vi "IR Opo Main.vi"() -> ()   [LabVIEW 2016] (continued)
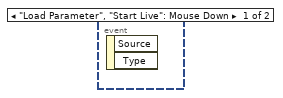
[diagram p2: hidden frame]
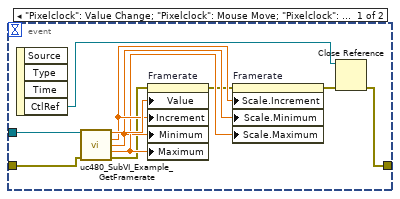
[diagram p3: hidden frame]
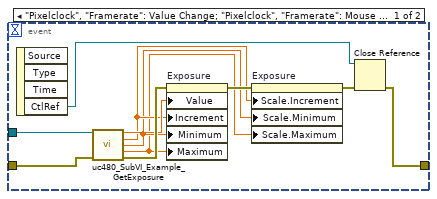
[diagram p4: hidden frame]
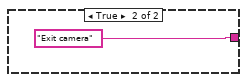
[diagram p5: hidden frame]
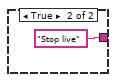
[diagram p6: hidden frame]
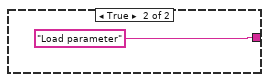
[diagram p7: hidden frame]
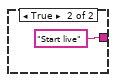
[diagram p8: hidden frame]
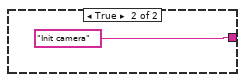
[diagram p9: hidden frame]
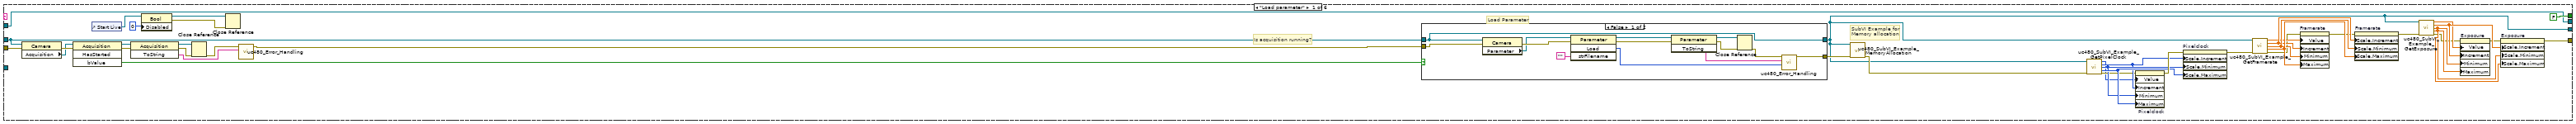
[diagram p10: hidden frame]
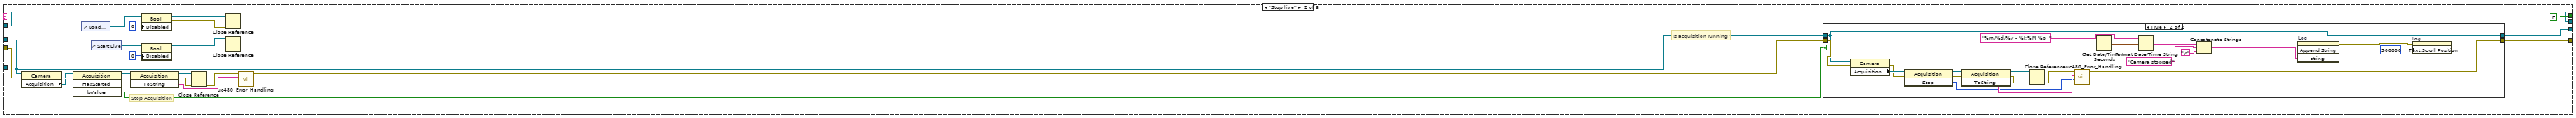
[diagram p12: hidden frame]
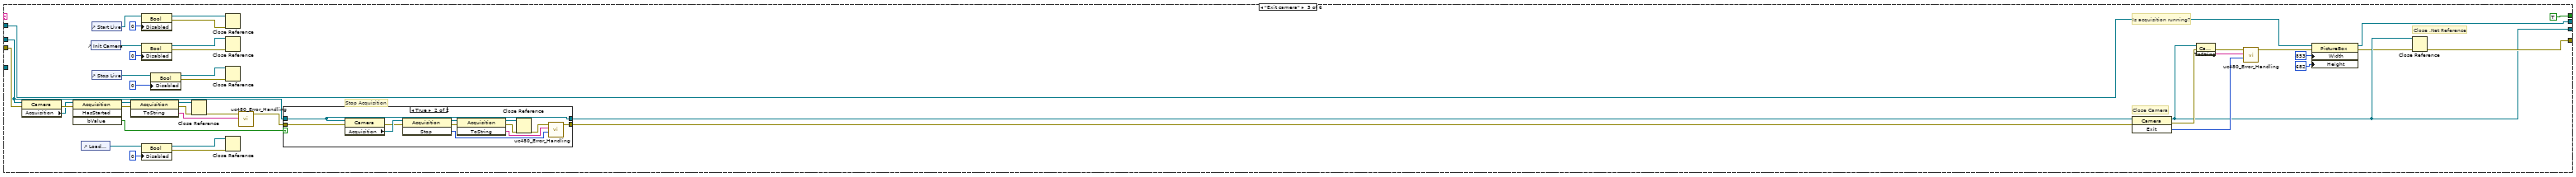
[diagram p14: hidden frame]
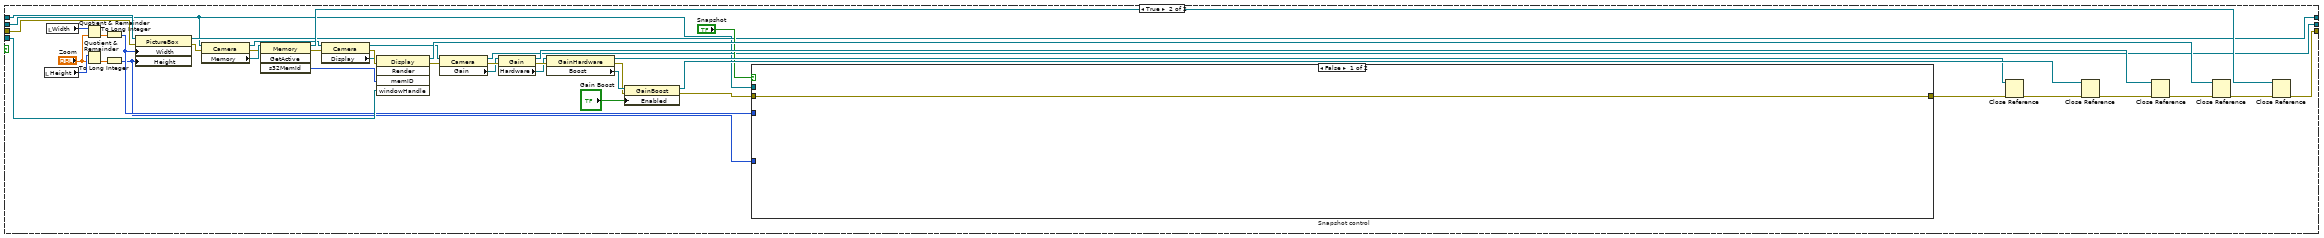
[diagram p16: hidden frame]
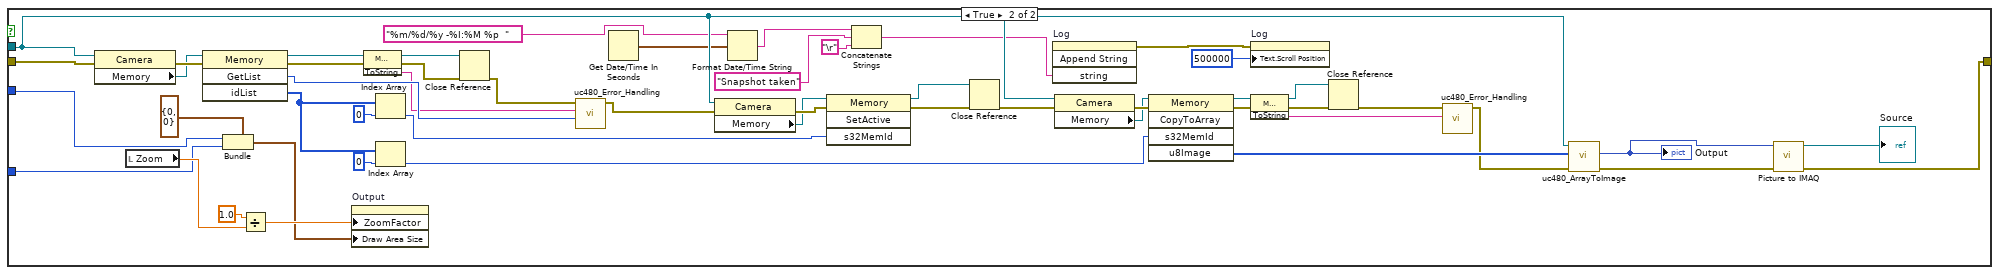
[diagram p17: hidden frame]
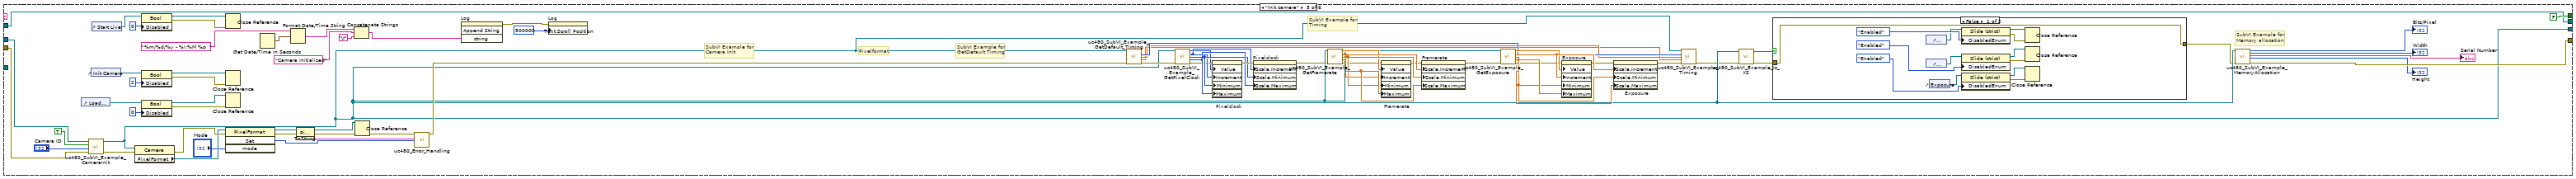
[diagram p18: hidden frame]
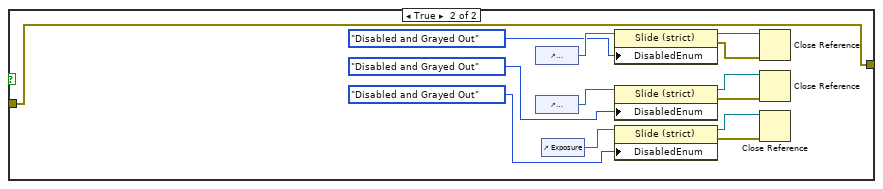
[diagram p19: hidden frame]
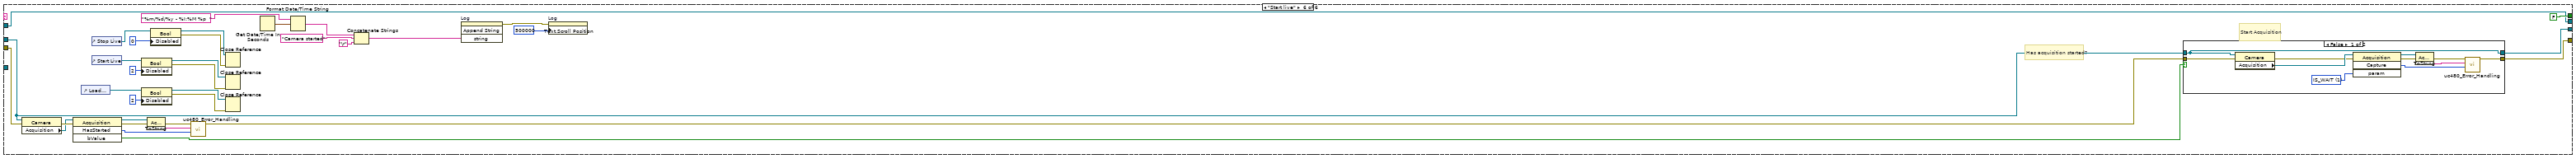
[diagram p20: hidden frame]
              frame False {
              }
              frame True {
                n542 = One Button Dialog(message="ATTENTION: you did not select\nany region of interest") -> ()  [unwired: 1 in, 1 out]
              }
            }
            n543 = local read "Heigth (µm)"() -> (w1034:i32)
            n544 = local read "Width (µm)"() -> (w1033:i32)
            n545 = Divide "X spot radius in micron"(x=w1033, y=w1028) -> (x/y=w1037:dbl)
            n546 = Divide "Y spot radius in micron"(x=w1034, y=w1028) -> (x/y=w1036:dbl)
            n547 = local read "Pixel size"() -> (w1002:dbl)
            n548 = Divide "X spot diameter in pixel"(x=w1033, y=w1002) -> (x/y=w1006:dbl)
            n549 = Divide "Y spot diameter in pixel"(x=w1034, y=w1002) -> (x/y=w1007:dbl)
            n550 = Multiply(x=w1002, y=w1002) -> (x*y=w1054:dbl)
            n551 = Multiply(x=w1070, y=w1002) -> (x*y=w1030:dbl)
            n552 = Multiply(x=w1069, y=w1002) -> (x*y=w1038:dbl)
            n553 = Round To Nearest(number=w1037) -> (nearest integer value=w1031:dbl)
            n554 = Round To Nearest(number=w1036) -> (nearest integer value=w1032:dbl)
            n555 = Add(x=w1030, y=w1031) -> (x+y=w1029:dbl)
            n556 = Add(x=w1038, y=w1032) -> (x+y=w1035:dbl)
            n557 = To Double Precision Float(number=w1049) -> (double precision float=w1052:dbl[][])
            n558 = Array Size(array=w1049) -> (size(s)=w1074:i32[])
            n559 = local read "Height  step \ndivider"() -> (w1076:i32)
            n560 = Divide(x=w1029, y=w1060) -> (x/y=w1062:dbl)
            n561 = Divide(x=w1035, y=w1060) -> (x/y=w1061:dbl)
            n562 = Add Array Elements(numeric array=w1052) -> (sum=w1056:dbl)
            n563 = Array To Cluster(array=w1074) -> (cluster=w1075:cluster{"[0]":i32, "[1]":i32})
            n564 = Number To Fractional String(number=w1062, precision (6)=w1068) -> (F-format string=w1047:string)  [unwired: 2 in]
            n565 = Number To Fractional String(number=w1061, precision (6)=w1068) -> (F-format string=w1048:string)  [unwired: 2 in]
            n566 = Unbundle(w1075) -> ("[0]"=w994:i32, "[1]"=w1010:i32)
            n567 = Divide(x=w1056, y=u8 255) -> (x/y=w1053:dbl)
            n568 = Multiply "# pixels in an ablation spot"(x=w1007, y=w1006) -> (x*y=w1009:dbl)
            n569 = Multiply(x=w1053, y=w1054) -> (x*y=w1044:dbl)
            n570 = Multiply(x=w994, y=w1002) -> (x*y=w1040:dbl)
            n571 = Multiply(x=w1010, y=w1002) -> (x*y=w1041:dbl)
            n572 = Subtract(x=w1010, y=w1006) -> (x-y=w1027:dbl)
            n573 = Fract/Exp String To Number(string=w1047) -> (number=→"Axis 1 Offset":dbl)  [unwired: 3 in, 1 out]
            n574 = Fract/Exp String To Number(string=w1048) -> (number=→"Axis 2 Offset":dbl)  [unwired: 3 in, 1 out]
            n575 = Divide "Height of a line"(x=w1007, y=w1076) -> (x/y=w1004:dbl)
            n576 = Divide "Total heigth lines"(x=w994, y=w1004) -> (x/y=w1008:dbl)
            n577 = Multiply(x=w1002, y=w1004) -> (x*y=w1005:dbl)
            n578 = Round To Nearest(number=w1040) -> (nearest integer value=→"ROI container\nheigth (µm)":dbl)
            n579 = Round To Nearest(number=w1041) -> (nearest integer value=→"ROI container\nwidth (µm)":dbl)
            n580 = Divide(x=w1044, y=1000000.0) -> (x/y=→"ROI Area \n(mm2)":dbl)
            n581 = Divide(x="Precision (%)", y=100.0) -> (x/y=w993:dbl)
            n582 = call "ROI parser.vi"("# pixels in an ablation spot"=w1009, "ROI Height in pixel"=w1008, "Heigth step size in pixel"=w1004, "ROI (8 bit image)"=w1049, "Ablation spot width"=w1006, "ROI Width in pixel"=w1027, "Sampling\nPrecision"=w993, "Ablation spot heigth"=w1007) -> ("Parsed array"=w1089:bool[][])  [unwired: 3 in]
            n583 = Index Array(array=w1089, index (col)=0 ("disabled index (col)")) -> (element=w1087:bool[])  [unwired: 1 in]
            n584 = Array Size(array=w1087) -> (size(s)=w1088:i32)
            n585 = call "Array processor.vi"("Source array"=w1089, "Iterations"=w1088) -> ("Lenght product array"=w1086:i32[][], "T/F product array"=w1023:bool[][])  [unwired: 8 in]
            n586 = for {
              tunnel: w1086 -> [w1099] mode=indexing
              tunnel: [w1098] -> w1072 mode=indexing
              tunnel: w1002 -> [w1097]
              # "This loop transform each lenght fragment into a µm size value"
              n587 = Multiply(x=w1097, y=w1099) -> (x*y=w1098:dbl[])
            }
            n588 = Array Size(array=w1023) -> (size(s)=w1022:i32[])
            n589 = Index Array(array=w1023, index (col)=0 ("disabled index (col)")) -> (element=w1078:bool[])  [unwired: 1 in]
            n590 = Array Size(array=w1078) -> (size(s)=w1077:i32)
            n591 = Index Array(array=w1022, index=0) -> (element=w1019:i32)
            n592 = Index Array(array=w1022, index=1) -> (element=w1018:i32)
            n593 = for {
              N: w1077 -> [_]
              tunnel: w1023 -> [w1096] mode=indexing
              tunnel: [w1094] -> w1059 mode=indexing
              # "This loop add a F for each Y moviment"
              n594 = Build Array (concatenate)(w1096, FALSE) -> (w1094:bool[])
            }
            "Laser on/off array" <- w1059
            n595 = Multiply(x=w1019, y=w1018) -> (x*y=w1017:i32)
            n596 = Multiply(x=w1017, y=w1016) -> (x*y=w1015:dbl)
            n597 = Round To Nearest(number=w1005) -> (nearest integer value=w1003:dbl)
            n598 = local read "Speed (µm/s)"() -> (w1024:i32)
            n599 = Index Array(array=w1072, index (col)=0 ("disabled index (col)")) -> (element=w1082:dbl[])  [unwired: 1 in]
            n600 = Index Array(array=w1072, index (row)=0) -> (element=w1084:dbl[])  [unwired: 1 in]
            n601 = Array Size(array=w1082) -> (size(s)=w1080:i32)
            n602 = Array Size(array=w1084) -> (size(s)=w1083:i32)
            n603 = local read "Axis 1"() -> (w1026:string)
            n604 = local read "Axis 2"() -> (w1025:string)
            n605 = call "Commands array generator.vi"("Axis 1"=w1026, "Heigth"=w1080, "Axis in"=w1025, "Width"=w1083, "Axes speed \n(µm/s)"=w1024, "Y Step size in µm"=w1003, "T/F product array"=w1023, "Space defined array"=w1072) -> ("Command Array"=→"Commands array":string[][], "Time Array"=w1039:dbl[][])  [unwired: 2 in]
            "Time array" <- w1039
            n606 = Add Array Elements(numeric array=w1039) -> (sum=w1014:dbl)
            n607 = Add(x=w1015, y=w1014) -> (x+y=w1013:dbl)
            "Processi time (sec)" <- w1013
            n608 = local write "Process time"(w1013) -> ()
          }
        }
      }
      event "Axes Manual Control": Value Change {
        n609 = event-data() -> ()  [unwired: 1 in, 6 out]
        n610 = case shown="True" "Axes Manual Control" {
          tunnel: w1102 -> [_ w1114]
          tunnel: w1101 -> [_ w1113]
          tunnel: w1100 -> [_ w1112]
          frame False {
          }
          frame True {
            n611 = flat-sequence {
              tunnel: w1114 -> [w1124]
              tunnel: w1113 -> [w1123]
              tunnel: w1112 -> [w1122]
              tunnel: [w1124] -> w1111
              tunnel: [w1123] -> w1110
              tunnel: [w1122] -> w1109
              tunnel: [w1121] -> w1108
              tunnel: [w1120] -> w1107
              tunnel: [w1119] -> w1106
              tunnel: [w1118] -> w1105
              tunnel: w1111 -> [w1167]
              tunnel: w1110 -> [w1166]
              tunnel: w1109 -> [w1165]
              tunnel: w1108 -> [w1160]
              tunnel: w1107 -> [w1159]
              tunnel: w1106 -> [w1150]
              tunnel: w1105 -> [w1149]
              frame #0 {
                n612 = call <userlib>:"Open TCP-IP.vi"("IP address"=w1124) -> ("error out"=w1116:errorcluster, "Connection ID"=w1125:T7)  [unwired: 8 in, 1 out]
                n613 = call <vilib>:"Simple Error Handler.vi"("error in (no error)"=w1116) -> ("error?"=w1115:bool, "error out"=w1117:errorcluster)  [unwired: 4 in, 3 out]
                n614 = case shown="True" w1115 {
                  tunnel: w1125 -> [w1140 _]
                  tunnel: w1117 -> [w1139 _]
                  tunnel: w1123 -> [w1136 _]
                  tunnel: w1122 -> [w1135 _]
                  tunnel: [w1134 w1144] -> w1121
                  tunnel: [w1133 w1144] -> w1120
                  tunnel: [w1129 w1143] -> w1119
                  tunnel: [w1128 w1143] -> w1118
                  frame False {
                    n615 = call "Get Stages Status.vi"("error in (no error)"=w1139, "Group Name (250 c max)"=w1136, "connection ID in"=w1140) -> ("error out"=w1138:errorcluster, "XPS error out"=w1137:errorcluster, "Group Status String"=w1133:string, "connection ID out"=w1132:T7, "Status"=w1128:i32)  [unwired: 4 in]
                    n616 = call "Get Stages Status.vi"("error in (no error)"=w1138, "XPS error in (no error)"=w1137, "Group Name (250 c max)"=w1135, "connection ID in"=w1132) -> ("error out"=w1142:errorcluster, "XPS error out"=w1131:errorcluster, "Group Status String"=w1134:string, "connection ID out"=w1141:T7, "Status"=w1129:i32)  [unwired: 3 in]
                    n617 = call <vilib>:"Simple Error Handler.vi"("error source (\" \")"="Axis manual control check" ("error source (\" \")"), "error in (no error)"=w1131) -> ()  [unwired: 3 in, 5 out]
                    n618 = call <userlib>:"Close TCP-IP.vi"("error in (no error)"=w1142, "connection ID in"=w1141) -> ("Error out"=w1130:errorcluster)  [unwired: 9 in]
                    n619 = call <vilib>:"Simple Error Handler.vi"("error source (\" \")"="TCP close Axis manual control check" ("error source (\" \")"), "error in (no error)"=w1130) -> ()  [unwired: 3 in, 5 out]
                  }
                  frame True {
                    w1143 = 0
                    w1144 = ""
                  }
                }
              }
              frame #1 {
                w1153 = 47 ("y")
                w1154 = "Ready"
                n620 = String Subset(string=w1159, offset (0)=0, length (rest)=5 ("length (rest)")) -> (substring=w1156:string)
                n621 = String Subset(string=w1160, offset (0)=0, length (rest)=5 ("length (rest)")) -> (substring=w1155:string)
                n622 = Equal?(x=w1156, y=w1154) -> (x = y?=w1157:bool)
                n623 = Equal?(x=w1154, y=w1155) -> (x = y?=w1158:bool)
                n624 = Equal?(x=w1153, y=w1149) -> (x = y?=w1151:bool)
                n625 = Equal?(x=w1150, y=w1153) -> (x = y?=w1152:bool)
                n626 = And(x=w1152, y=w1151) -> (x .and. y?=w1146:bool)
                n627 = And(x=w1157, y=w1158) -> (x .and. y?=w1147:bool)
                n628 = Not(x=w1146) -> (.not. x?=w1145:bool)
                n629 = And(x=w1147, y=w1145) -> (x .and. y?=w1148:bool)
                n630 = case shown="True" w1148 {
                  tunnel: w1167 -> [_ w1173]
                  tunnel: w1166 -> [_ w1172]
                  tunnel: w1165 -> [_ w1171]
                  tunnel: w1145 -> [w1168 _]
                  frame False {
                    n631 = case shown="False" w1168 {
                      frame False {
                        n632 = One Button Dialog(message="One or more axis already in jogging position") -> ()  [unwired: 1 in, 1 out]
                      }
                      frame True {
                        n633 = One Button Dialog(message="Axes are not ready") -> ()  [unwired: 1 in, 1 out]
                      }
                    }
                  }
                  frame True {
                    n634 = call "XPS_LTA_HS_Jogger.vi"("Axis 2"=w1171, "Axis 1"=w1172, "Controller Address"=w1173) -> ()  [unwired: 8 in]
                  }
                }
              }
            }
          }
        }
      }
      event "Home Axes": Value Change {
        n635 = event-data() -> ()  [unwired: 1 in, 6 out]
        n636 = flat-sequence {
          tunnel: w1180 -> [w1186]
          tunnel: w1181 -> [w1187]
          tunnel: w1182 -> [w1188]
          tunnel: "Home Axes" -> [w1189]
          tunnel: [w1189] -> w1178
          tunnel: [w1188] -> w1177
          tunnel: [w1187] -> w1176
          tunnel: [w1186] -> w1175
          tunnel: [w1185] -> w1174
          tunnel: [w1193] -> w1179
          tunnel: w1178 -> [w1191]
          tunnel: w1177 -> [w1196]
          tunnel: w1176 -> [w1194]
          tunnel: w1175 -> [w1195]
          tunnel: w1174 -> [w1192]
          tunnel: [w1275] -> w1183
          tunnel: w1179 -> [w1274]
          frame #0 {
            n637 = call "Display Message to User"() -> ("OK"=w1185:bool)  [unwired: 10 in, 1 out]
          }
          frame #1 {
            n638 = And(x=w1191, y=w1192) -> (x .and. y?=w1190:bool)
            n639 = case shown="True" w1190 {
              tunnel: w1196 -> [_ w1212]
              tunnel: w1194 -> [_ w1213]
              tunnel: w1195 -> [_ w1210]
              tunnel: w1194 -> [_ w1211]
              tunnel: [FALSE w1203] -> w1193
              frame False {
              }
              frame True {
                w1209 = 47 ("y")
                w1225 = "Ready"
                n640 = call <userlib>:"Open TCP-IP.vi"("IP address"=w1212) -> ("error out"=w1198:errorcluster, "Connection ID"=w1216:T7)  [unwired: 8 in, 1 out]
                n641 = call <vilib>:"Simple Error Handler.vi"("error in (no error)"=w1198) -> ("error?"=w1200:bool, "error out"=w1199:errorcluster)  [unwired: 4 in, 3 out]
                n642 = case shown="True" w1200 {
                  tunnel: w1199 -> [w1239 _]
                  tunnel: w1216 -> [w1238 _]
                  tunnel: [w1235 w1244] -> w1215
                  tunnel: [w1234 w1244] -> w1214
                  tunnel: w1213 -> [w1233 _]
                  tunnel: w1210 -> [w1232 _]
                  tunnel: [w1229 w1243] -> w1208
                  tunnel: [w1228 w1243] -> w1207
                  frame False {
                    n643 = call "Get Stages Status.vi"("error in (no error)"=w1239, "Group Name (250 c max)"=w1233, "connection ID in"=w1238) -> ("error out"=w1240:errorcluster, "XPS error out"=w1241:errorcluster, "Group Status String"=w1235:string, "connection ID out"=w1242:T7, "Status"=w1228:i32)  [unwired: 4 in]
                    n644 = call "Get Stages Status.vi"("error in (no error)"=w1240, "XPS error in (no error)"=w1241, "Group Name (250 c max)"=w1232, "connection ID in"=w1242) -> ("error out"=w1236:errorcluster, "XPS error out"=w1231:errorcluster, "Group Status String"=w1234:string, "connection ID out"=w1237:T7, "Status"=w1229:i32)  [unwired: 3 in]
                    n645 = call <vilib>:"Simple Error Handler.vi"("error source (\" \")"="home axis check" ("error source (\" \")"), "error in (no error)"=w1231) -> ()  [unwired: 3 in, 5 out]
                    n646 = call <userlib>:"Close TCP-IP.vi"("error in (no error)"=w1236, "connection ID in"=w1237) -> ("Error out"=w1230:errorcluster)  [unwired: 9 in]
                    n647 = call <vilib>:"Simple Error Handler.vi"("error source (\" \")"="TCP close home axis check" ("error source (\" \")"), "error in (no error)"=w1230) -> ()  [unwired: 3 in, 5 out]
                  }
                  frame True {
                    w1243 = 0
                    w1244 = ""
                  }
                }
                n648 = Equal?(x=w1209, y=w1207) -> (x = y?=w1206:bool)
                n649 = Equal?(x=w1208, y=w1209) -> (x = y?=w1205:bool)
                n650 = String Subset(string=w1215, offset (0)=0, length (rest)=5 ("length (rest)")) -> (substring=w1223:string)
                n651 = String Subset(string=w1214, offset (0)=0, length (rest)=5 ("length (rest)")) -> (substring=w1224:string)
                n652 = Equal?(x=w1223, y=w1225) -> (x = y?=w1222:bool)
                n653 = Equal?(x=w1225, y=w1224) -> (x = y?=w1221:bool)
                n654 = And(x=w1205, y=w1206) -> (x .and. y?=w1201:bool)
                n655 = Not(x=w1201) -> (.not. x?=w1202:bool)
                n656 = And(x=w1222, y=w1221) -> (x .and. y?=w1204:bool)
                n657 = And(x=w1204, y=w1202) -> (x .and. y?=w1203:bool)
                n658 = case shown="True" w1203 {
                  tunnel: w1212 -> [_ w1254]
                  tunnel: w1211 -> [_ w1253]
                  tunnel: w1210 -> [_ w1252]
                  tunnel: w1201 -> [w1245 _]
                  frame False {
                    n659 = case shown="True" w1245 {
                      frame False {
                        n660 = One Button Dialog(message="Axes are not ready") -> ()  [unwired: 1 in, 1 out]
                      }
                      frame True {
                        n661 = One Button Dialog(message="One or more axis are in jogging mode") -> ()  [unwired: 1 in, 1 out]
                      }
                    }
                  }
                  frame True {
                    n662 = call <userlib>:"Open TCP-IP.vi"("IP address"=w1254) -> ("error out"=w1270:errorcluster, "Connection ID"=w1271:T7)  [unwired: 8 in, 1 out]
                    n663 = call <userlib>:"Group Kill.vi"("error in (no error)"=w1270, "Group Name (250 c max)"=w1253, "connection ID in"=w1271) -> ("error out"=w1268:errorcluster, "XPS error out"=w1269:errorcluster, "connection ID out"=w1265:T7)  [unwired: 6 in]
                    n664 = call <userlib>:"Group Initialize.vi"("error in (no error)"=w1268, "XPS error in (no error)"=w1269, "Group Name (250 c max)"=w1253, "connection ID in"=w1265) -> ("error out"=w1266:errorcluster, "XPS error out"=w1267:errorcluster, "connection ID out"=w1264:T7)  [unwired: 5 in]
                    n665 = call <userlib>:"Group Home Search.vi"("error in (no error)"=w1266, "XPS error in (no error)"=w1267, "Group Name (250 c max)"=w1253, "connection ID in"=w1264) -> ("error out"=w1255:errorcluster, "XPS error out"=w1256:errorcluster, "connection ID out"=w1263:T7)  [unwired: 5 in]
                    n666 = call <userlib>:"Group Kill.vi"("error in (no error)"=w1255, "XPS error in (no error)"=w1256, "Group Name (250 c max)"=w1252, "connection ID in"=w1263) -> ("error out"=w1257:errorcluster, "XPS error out"=w1258:errorcluster, "connection ID out"=w1262:T7)  [unwired: 5 in]
                    n667 = call <userlib>:"Group Initialize.vi"("error in (no error)"=w1257, "XPS error in (no error)"=w1258, "Group Name (250 c max)"=w1252, "connection ID in"=w1262) -> ("error out"=w1259:errorcluster, "XPS error out"=w1260:errorcluster, "connection ID out"=w1261:T7)  [unwired: 5 in]
                    n668 = call <userlib>:"Group Home Search.vi"("error in (no error)"=w1259, "XPS error in (no error)"=w1260, "Group Name (250 c max)"=w1252, "connection ID in"=w1261) -> ("error out"=w1272:errorcluster, "XPS error out"=w1251:errorcluster, "connection ID out"=w1273:T7)  [unwired: 5 in]
                    n669 = call <vilib>:"Simple Error Handler.vi"("error source (\" \")"="home axis " ("error source (\" \")"), "error in (no error)"=w1251) -> ()  [unwired: 3 in, 5 out]
                    n670 = call <userlib>:"Close TCP-IP.vi"("error in (no error)"=w1272, "connection ID in"=w1273) -> ("Error out"=w1250:errorcluster)  [unwired: 9 in]
                    n671 = call <vilib>:"Simple Error Handler.vi"("error source (\" \")"="TCP close home axis " ("error source (\" \")"), "error in (no error)"=w1250) -> ()  [unwired: 3 in, 5 out]
                  }
                }
              }
            }
          }
          frame #2 {
            n672 = case shown="True" w1274 {
              tunnel: ["" ("StringOut") "Axes have been moved to home position" ("StringOut")] -> w1275
              frame False {
              }
              frame True {
              }
            }
          }
        }
      }
      event "Transparency": Value Change {
        n673 = event-data() -> ()  [unwired: 1 in, 6 out]
        n674 = control-ref of="This VI"() -> (w1279:refnum<vi>)
        n675 = property class="VI"(reference=w1279, "FP:Transparency"="Transparency") -> ()  [unwired: 1 in, 2 out]
      }
      event "Capture": Value Change {
        w1290 = 47 ("y")
        w1306 = "Ready"
        n676 = event-data() -> ()  [unwired: 1 in, 6 out]
        n677 = call <userlib>:"Open TCP-IP.vi"("IP address"=w1294) -> ("error out"=w1282:errorcluster, "Connection ID"=w1297:T7)  [unwired: 8 in, 1 out]
        n678 = call <vilib>:"Simple Error Handler.vi"("error in (no error)"=w1282) -> ("error?"=w1280:bool, "error out"=w1281:errorcluster)  [unwired: 4 in, 3 out]
        n679 = case shown="True" w1280 {
          tunnel: w1281 -> [w1320 _]
          tunnel: w1297 -> [w1319 _]
          tunnel: [w1316 w1324] -> w1296
          tunnel: [w1315 w1324] -> w1295
          tunnel: w1293 -> [w1314 _]
          tunnel: w1292 -> [w1313 _]
          tunnel: [w1311 w1325] -> w1291
          tunnel: [w1310 w1325] -> w1289
          frame False {
            n680 = call "Get Stages Status.vi"("error in (no error)"=w1320, "Group Name (250 c max)"=w1314, "connection ID in"=w1319) -> ("error out"=w1321:errorcluster, "XPS error out"=w1322:errorcluster, "Group Status String"=w1316:string, "connection ID out"=w1323:T7, "Status"=w1310:i32)  [unwired: 4 in]
            n681 = call "Get Stages Status.vi"("error in (no error)"=w1321, "XPS error in (no error)"=w1322, "Group Name (250 c max)"=w1313, "connection ID in"=w1323) -> ("error out"=w1317:errorcluster, "XPS error out"=w1312:errorcluster, "Group Status String"=w1315:string, "connection ID out"=w1318:T7, "Status"=w1311:i32)  [unwired: 3 in]
            n682 = call <vilib>:"Simple Error Handler.vi"("error source (\" \")"="Capture check" ("error source (\" \")"), "error in (no error)"=w1312) -> ()  [unwired: 3 in, 5 out]
            n683 = call <userlib>:"Close TCP-IP.vi"("error in (no error)"=w1317, "connection ID in"=w1318) -> ("Error out"=w1308:errorcluster)  [unwired: 9 in]
            n684 = call <vilib>:"Simple Error Handler.vi"("error in (no error)"=w1308) -> ()  [unwired: 4 in, 5 out]
          }
          frame True {
            w1325 = 0
            w1324 = ""
          }
        }
        n685 = Equal?(x=w1290, y=w1289) -> (x = y?=w1287:bool)
        n686 = Equal?(x=w1291, y=w1290) -> (x = y?=w1288:bool)
        n687 = String Subset(string=w1296, offset (0)=0, length (rest)=5 ("length (rest)")) -> (substring=w1304:string)
        n688 = String Subset(string=w1295, offset (0)=0, length (rest)=5 ("length (rest)")) -> (substring=w1305:string)
        n689 = Equal?(x=w1304, y=w1306) -> (x = y?=w1303:bool)
        n690 = Equal?(x=w1306, y=w1305) -> (x = y?=w1302:bool)
        n691 = And(x=w1288, y=w1287) -> (x .and. y?=w1284:bool)
        n692 = And(x=w1303, y=w1302) -> (x .and. y?=w1286:bool)
        n693 = Not(x=w1284) -> (.not. x?=w1283:bool)
        n694 = And(x=w1286, y=w1283) -> (x .and. y?=w1285:bool)
        n695 = case shown="True" w1285 {
          tunnel: ["" w1333] -> w1307
          tunnel: w1294 -> [_ w1332]
          tunnel: w1292 -> [_ w1331]
          tunnel: w1293 -> [_ w1330]
          tunnel: w1284 -> [w1326 _]
          frame False {
            n696 = case shown="True" w1326 {
              frame False {
                n697 = One Button Dialog(message="Axes are not ready") -> ()  [unwired: 1 in, 1 out]
              }
              frame True {
                n698 = One Button Dialog(message="One or more axis are in jogging mode") -> ()  [unwired: 1 in, 1 out]
              }
            }
          }
          frame True {
            n699 = flat-sequence {
              tunnel: [w1354] -> w1345
              tunnel: [w1353] -> w1344
              tunnel: [w1352] -> w1343
              tunnel: [w1351] -> w1342
              tunnel: [w1350] -> w1341
              tunnel: [w1349] -> w1340
              tunnel: [w1348] -> w1339
              tunnel: w1332 -> [w1348]
              tunnel: w1331 -> [w1347]
              tunnel: w1330 -> [w1346]
              tunnel: w1345 -> [w1374]
              tunnel: w1344 -> [w1365]
              tunnel: w1343 -> [w1366]
              tunnel: w1342 -> [w1372]
              tunnel: w1341 -> [w1371]
              tunnel: [w1364] -> w1338
              tunnel: w1340 -> [w1364]
              tunnel: [w1363] -> w1337
              tunnel: w1339 -> [w1363]
              tunnel: [w1376] -> w1336
              tunnel: w1338 -> [w1376]
              tunnel: [w1375] -> w1335
              tunnel: w1337 -> [w1375]
              tunnel: w1336 -> [w1382]
              tunnel: w1335 -> [w1387]
              tunnel: [w1381] -> w1334
              tunnel: [w1397] -> w1333
              tunnel: w1334 -> [w1394]
              frame #0 {
                w1359 = ".Pos"
                n700 = local read "Axis Initial Parameters"() -> (w1349:T1)
                n701 = Concatenate Strings(w1346, w1359) -> (w1353:string)
                n702 = call <userlib>:"Open TCP-IP.vi"("IP address"=w1348) -> ("error out"=w1355:errorcluster, "Connection ID"=w1360:T7)  [unwired: 5 in, 4 out]
                n703 = call <userlib>:"Positioner SGamma Parameters Set.vi"("SGamma Parameters"=w1349, "error in (no error)"=w1355, "Positioner Name (250 c max)"=w1353, "connection ID in"=w1360) -> ("error out"=w1356:errorcluster, "XPS error out"=w1357:errorcluster, "connection ID out"=w1358:T7)  [unwired: 5 in]
                n704 = Concatenate Strings(w1347, w1359) -> (w1352:string)
                n705 = call <userlib>:"Positioner SGamma Parameters Set.vi"("SGamma Parameters"=w1349, "error in (no error)"=w1356, "XPS error in (no error)"=w1357, "Positioner Name (250 c max)"=w1352, "connection ID in"=w1358) -> ("error out"=w1351:errorcluster, "XPS error out"=w1350:errorcluster, "connection ID out"=w1354:T7)  [unwired: 4 in]
              }
              frame #1 {
                n706 = local read "Axis 2 Offset"() -> (w1362:dbl)
                n707 = local read "Axis 1 Offset"() -> (w1361:dbl)
                n708 = call <userlib>:"Single Axis Group Move Relative.vi"("Target Displacement (units)"=w1362, "error in (no error)"=w1372, "XPS error in (no error)"=w1371, "SingleAxis Group  Name (250 c max)"=w1365, "connection ID in"=w1374) -> ("error out"=w1369:errorcluster, "XPS error out"=w1370:errorcluster, "connection ID out"=w1373:T7)  [unwired: 4 in]
                n709 = call <userlib>:"Single Axis Group Move Relative.vi"("Target Displacement (units)"=w1361, "error in (no error)"=w1369, "XPS error in (no error)"=w1370, "SingleAxis Group  Name (250 c max)"=w1366, "connection ID in"=w1373) -> ("error out"=w1367:errorcluster, "connection ID out"=w1368:T7)  [unwired: 4 in, 1 out]
                n710 = call <userlib>:"Close TCP-IP.vi"("error in (no error)"=w1367, "connection ID in"=w1368) -> ()  [unwired: 9 in, 1 out]
              }
              frame #2 {
                n711 = Wait (ms)(milliseconds to wait=u32 1000) -> ()  [unwired: 1 out]
              }
              frame #3 {
                n712 = local read "Speed (µm/s)"() -> (w1386:i32)
                n713 = local read "Processi time (sec)"() -> (w1380:i32)
                n714 = local read "Laser on/off array"() -> (w1391:bool[][])
                n715 = local read "Commands array"() -> (w1392:string[][])
                n716 = local read "Alignment \ndiode"() -> (w1390:bool)
                n717 = local read "ROI Area \n(mm2)"() -> (w1378:dbl)
                n718 = Divide(x=w1386, y=1000) -> (x/y=w1383:dbl)
                n719 = call "IR_OPO_Capture_V2.vi"("Commands array"=w1392, "Laser on/off array"=w1391, "AD status"=w1390, "XPS_Address"=w1387, "laser array index"=0, "OPO on?"=TRUE, "Process time"=w1380, "Axis Speed"=w1383, "stop"=FALSE ("STOP CAPTURE"), "Axis Initial Parameters"=w1382, "ROI Area \n(mm2)"=w1378, "Acceleration (units/seconds²)"="Acceleration \n(mm/s²)") -> ("Elapsed time"=w1381:dbl)  [unwired: 3 in]
              }
              frame #4 {
                n720 = Number To Decimal String(number=w1394) -> (decimal integer string=w1393:string)  [unwired: 1 in]
                n721 = Concatenate Strings("Capture completed in " ("StringOut"), w1393, " seconds" ("string")) -> (w1397:string)
              }
            }
          }
        }
      }
    }
    n722 = Get Date/Time In Seconds() -> (seconds since 1Jan1904=w758:timestamp)
    n723 = Format Date/Time String(time format string (%c)="%m/%d/%y - %I:%M %p  ", seconds (now)=w758) -> (date/time string=w757:string)  [unwired: 1 in]
    n724 = Empty String/Path?(string/path=w754) -> (empty?=w756:bool)
    n725 = Concatenate Strings(w757, w754, "\r") -> (w755:string)
    n726 = case shown="False" w756 {
      tunnel: w755 -> [w764 _]
      frame False {
        n727 = invoke on="Log" class="Str" method="Append String"("string"=w764) -> (error out=w763:errorcluster)  [unwired: 3 in, 3 out]
        n728 = property on="Log" class="Str"(error in=w763, "Text.Scroll Position"=u32 500000) -> ()  [unwired: 1 in, 2 out]
      }
      frame True {
      }
    }
  }
  n729 = control-ref of="Init Camera"() -> (w45:refnum<vi>)
  n730 = control-ref of="Stop Live"() -> (w38:refnum<vi>)
  n731 = property class="Bool"(reference=w38, "Disabled"=u8 2 ("Deaktiviert")) -> (reference out=w29:refnum<vi>, error out=w28:errorcluster)  [unwired: 1 in]
  n732 = property class="Bool"(reference=w45, "Disabled"=u8 0 ("Deaktiviert")) -> (reference out=w33:refnum<vi>, error out=w32:errorcluster)  [unwired: 1 in]
  n733 = Close Reference(reference=w29, error in (no error)=w28) -> ()  [unwired: 1 out]
  n734 = Close Reference(reference=w33, error in (no error)=w32) -> ()  [unwired: 1 out]
  n735 = control-ref of="Load Parameter"() -> (w39:refnum<vi>)
  n736 = control-ref of="Start Live"() -> (w42:refnum<vi>)
  n737 = property class="Bool"(reference=w42, "Disabled"=u8 2 ("Deaktiviert")) -> (reference out=w31:refnum<vi>, error out=w30:errorcluster)  [unwired: 1 in]
  n738 = property class="Bool"(reference=w39, "Disabled"=u8 2 ("Deaktiviert")) -> (reference out=w27:refnum<vi>, error out=w26:errorcluster)  [unwired: 1 in]
  n739 = Close Reference(reference=w31, error in (no error)=w30) -> ()  [unwired: 1 out]
  n740 = Close Reference(reference=w27, error in (no error)=w26) -> ()  [unwired: 1 out]
